vi "Read Audio File (Polymorphic Template).vi"   [LabVIEW 2020]
uses:
  06e8507e-5cc6-4715-b89b-25d08780c2c3.vi
  10b2a4eb-5bd8-4a2d-b853-82183560208b.vi
  5a0112e6-620d-4b69-8fed-8155b5fad54c.vi
  7ceaf824-825f-4488-b6f6-58092615eaee.vi
  e85dd151-54ad-4fd7-ba3f-92fd74706804.vi
  bb12b8a1-e9b4-444a-8006-34dff706d250.vi
  248f0d84-3123-4200-a913-bcfea1f68da1.vi
  8d061356-47c1-4895-9c6f-99d6d71e1bec.vi
  e334dc1d-1e69-47d0-9aa9-295499adad90.vi
  7bf0e060-53cf-452d-bbea-fc881f6a4cc3.vi
  356f7f25-4a52-45fa-8418-8a7bd3d76278.vi
  3ef80b9f-cd16-44e5-98c1-505e395ad75f.vi
  a1416795-6e25-46b3-a9be-8e6cfc0fe23c.vi
  ff9dc6f9-be12-46b6-b368-308dd6c8875e.vi
  d165e2c0-5d31-4aab-88ec-8d6b30ad1ee5.vi
  0d93b7bc-de39-4a9a-bece-77059c55d397.vi
  ccc2c4b2-55b1-46cc-9dda-dcb11ac68a7f.vi
  7f73cb6f-fdb3-4d0b-bdd3-0057334248ea.vi
  4781f742-4336-4a42-965d-a1c1c91b1209.vi
  c0b0459d-b72a-4581-a6dd-fd2eb5f8281e.vi
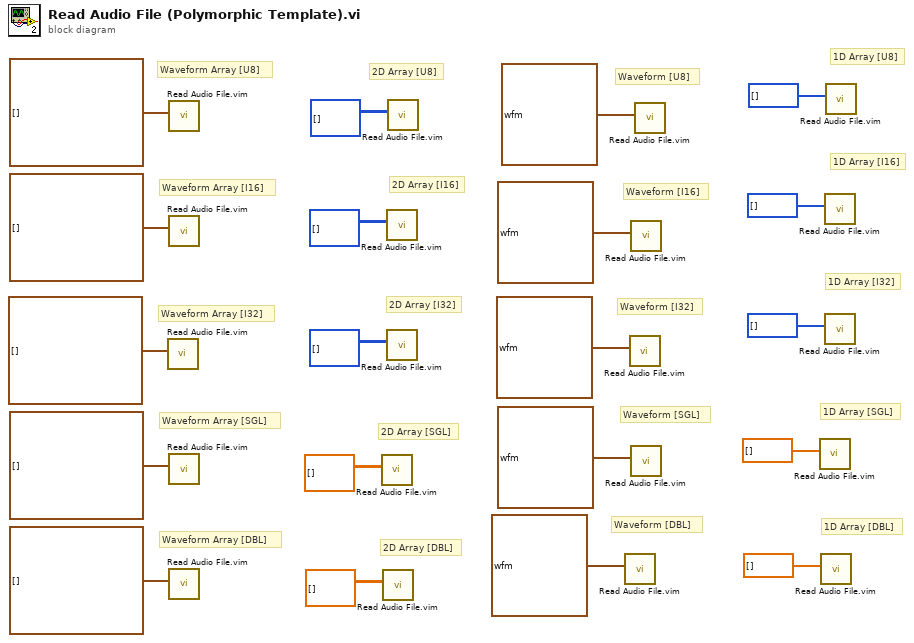
[diagram p0: block diagram]
diagram:
  # "1D Array [DBL]"
  # "1D Array [SGL]"
  # "1D Array [I32]"
  # "1D Array [I16]"
  # "1D Array [U8]"
  # "Waveform [DBL]"
  # "Waveform [SGL]"
  # "Waveform [I32]"
  # "Waveform [I16]"
  # "Waveform [U8]"
  # "2D Array [DBL]"
  # "2D Array [SGL]"
  # "2D Array [I32]"
  # "2D Array [I16]"
  # "2D Array [U8]"
  # "Waveform Array [DBL]"
  # "Waveform Array [SGL]"
  # "Waveform Array [I32]"
  # "Waveform Array [I16]"
  # "Waveform Array [U8]"
  n1 = call "Read Audio File.vim"("Data Format"=waveform(i32)[] [] ("Data Format (I16 Waveform Array)")) -> ()  [unwired: 6 in, 5 out]
  n2 = call "Read Audio File.vim"("Data Format"=waveform(u8)[] [] ("Data Format (I16 Waveform Array)")) -> ()  [unwired: 6 in, 5 out]
  n3 = call "Read Audio File.vim"("Data Format"=waveform(i16)[] [] ("Data Format (I16 Waveform Array)")) -> ()  [unwired: 6 in, 5 out]
  n4 = call "Read Audio File.vim"("Data Format"=waveform(sgl)[] [] ("Data Format (I16 Waveform Array)")) -> ()  [unwired: 6 in, 5 out]
  n5 = call "Read Audio File.vim"("Data Format"=waveform(dbl)[] [] ("Data Format (I16 Waveform Array)")) -> ()  [unwired: 6 in, 5 out]
  n6 = call "Read Audio File.vim"("Data Format"=sgl[][] []) -> ()  [unwired: 6 in, 5 out]
  n7 = call "Read Audio File.vim"("Data Format"=dbl[][] []) -> ()  [unwired: 6 in, 5 out]
  n8 = call "Read Audio File.vim"("Data Format"=i16[][] []) -> ()  [unwired: 6 in, 5 out]
  n9 = call "Read Audio File.vim"("Data Format"=i32[][] []) -> ()  [unwired: 6 in, 5 out]
  n10 = call "Read Audio File.vim"("Data Format"=u8[][] []) -> ()  [unwired: 6 in, 5 out]
  n11 = call "Read Audio File.vim"("Data Format"=waveform(dbl) {"t0"=timestamp(0 s since 1904-01-01), "dt"=1.0, "Y"=[]} ("Waveform")) -> ()  [unwired: 6 in, 5 out]
  n12 = call "Read Audio File.vim"("Data Format"=waveform(i32) {"t0"=timestamp(0 s since 1904-01-01), "dt"=1.0, "Y"=[]} ("Waveform")) -> ()  [unwired: 6 in, 5 out]
  n13 = call "Read Audio File.vim"("Data Format"=waveform(i16) {"t0"=timestamp(0 s since 1904-01-01), "dt"=1.0, "Y"=[]} ("Waveform")) -> ()  [unwired: 6 in, 5 out]
  n14 = call "Read Audio File.vim"("Data Format"=waveform(sgl) {"t0"=timestamp(0 s since 1904-01-01), "dt"=1.0, "Y"=[]} ("Waveform")) -> ()  [unwired: 6 in, 5 out]
  n15 = call "Read Audio File.vim"("Data Format"=waveform(u8) {"t0"=timestamp(0 s since 1904-01-01), "dt"=1.0, "Y"=[]} ("Waveform")) -> ()  [unwired: 6 in, 5 out]
  n16 = call "Read Audio File.vim"("Data Format"=sgl[] []) -> ()  [unwired: 6 in, 5 out]
  n17 = call "Read Audio File.vim"("Data Format"=dbl[] []) -> ()  [unwired: 6 in, 5 out]
  n18 = call "Read Audio File.vim"("Data Format"=i16[] []) -> ()  [unwired: 6 in, 5 out]
  n19 = call "Read Audio File.vim"("Data Format"=i32[] []) -> ()  [unwired: 6 in, 5 out]
  n20 = call "Read Audio File.vim"("Data Format"=u8[] []) -> ()  [unwired: 6 in, 5 out]
